vi "Frog generate Simu.vi"() -> ()   [LabVIEW 2024, in "File manipulate.lvclass"]
uses:
  File manipulate.lvclass
  File manipulate.lvclass/File manipulate.ctl
panel:
  in  "Transpose FROG Trace":bool
  out "temporal phase":cluster{"Y":dbl[], "Y":dbl[]}[](graph)
  in  "Save Fichier":bool
  in  "dispersive element":T1={"material"="BK7", "thickness"=0.0} {"thickness" format="%.2f"}
  out "Lambda":dbl[](array[numeric])=[479.83343142647254, 480.4599804843464, 481.0865295422202, 481.71307860009404, 482.33962765796787, 482.9661767158417, 483.59272577371553, 484.21927483158936, 484.8458238894632, 485.472372947337, 486.09892200521085, 486.7254710630847, 487.3520201209585, 487.97856917883234, 488.6051182367062, 489.23166729458, 489.85821635245384, 490.48476541032767, 491.1113144682015, 491.73786352607533, 492.36441258394916, 492.990961641823, 493.6175106996968, 494.24405975757065, 494.8706088154445, 495.4971578733183, 496.12370693119215, 496.750255989066, 497.3768050469398, 498.00335410481364, 498.62990316268747, 499.2564522205613, 499.88300127843513, 500.50955033630896, 501.1360993941828, 501.7626484520566, 502.38919750993045, 503.0157465678043, 503.6422956256781, 504.26884468355195, 504.8953937414258, 505.5219427992996, 506.14849185717344, 506.77504091504727, 507.4015899729211, 508.02813903079493, 508.65468808866876, 509.2812371465426, 509.9077862044164, 510.53433526229026, 511.1608843201641, 511.7874333780379, 512.4139824359117, 513.0405314937856, 513.6670805516594, 514.2936296095332, 514.9201786674071, 515.5467277252809, 516.1732767831547, 516.7998258410286, 517.4263748989024, 518.0529239567762, 518.6794730146501, 519.3060220725239, 519.9325711303977, 520.5591201882715, 521.1856692461454, 521.8122183040192, 522.438767361893, 523.0653164197669, 523.6918654776407, 524.3184145355145, 524.9449635933884, 525.5715126512622, 526.198061709136, 526.8246107670099, 527.4511598248837, 528.0777088827575, 528.7042579406314, 529.3308069985052, 529.957356056379, 530.5839051142528, 531.2104541721267, 531.8370032300005, 532.4635522878743, 533.0901013457482, 533.716650403622, 534.3431994614958, 534.9697485193697, 535.5962975772435, 536.2228466351173, 536.8493956929912, 537.475944750865, 538.1024938087388, 538.7290428666126, 539.3555919244865, 539.9821409823603, 540.6086900402341, 541.235239098108, 541.8617881559818, 542.4883372138556, 543.1148862717295, 543.7414353296033, 544.3679843874771, 544.994533445351, 545.6210825032248, 546.2476315610986, 546.8741806189724, 547.5007296768463, 548.1272787347201, 548.7538277925939, 549.3803768504678, 550.0069259083416, 550.6334749662154, 551.2600240240893, 551.8865730819631, 552.5131221398369, 553.1396711977108, 553.7662202555846, 554.3927693134584, 555.0193183713322, 555.6458674292061, 556.2724164870799, 556.8989655449537, 557.5255146028276, 558.1520636607014, 558.7786127185752, 559.4051617764491, 560.0317108343229, 560.6582598921967, 561.2848089500706, 561.9113580079444, 562.5379070658182, 563.164456123692, 563.7910051815659, 564.4175542394397, 565.0441032973135, 565.6706523551874, 566.2972014130612, 566.923750470935, 567.5502995288089, 568.1768485866827, 568.8033976445565, 569.4299467024304, 570.0564957603042, 570.683044818178, 571.3095938760518, 571.9361429339257, 572.5626919917995, 573.1892410496733, 573.8157901075472, 574.442339165421, 575.0688882232948, 575.6954372811687, 576.3219863390425, 576.9485353969163, 577.5750844547902, 578.201633512664, 578.8281825705378, 579.4547316284117, 580.0812806862855, 580.7078297441593, 581.3343788020331, 581.960927859907, 582.5874769177808, 583.2140259756546, 583.8405750335285, 584.4671240914023, 585.0936731492761, 585.72022220715, 586.3467712650238, 586.9733203228976, 587.5998693807715, 588.2264184386453, 588.8529674965191, 589.479516554393, 590.1060656122668, 590.7326146701406, 591.3591637280144, 591.9857127858883, 592.6122618437621, 593.2388109016359, 593.8653599595098, 594.4919090173836, 595.1184580752574, 595.7450071331313, 596.3715561910051, 596.9981052488789, 597.6246543067527, 598.2512033646266, 598.8777524225004, 599.5043014803742, 600.1308505382481, 600.7573995961219, 601.3839486539957, 602.0104977118696, 602.6370467697434, 603.2635958276172, 603.890144885491, 604.5166939433649, 605.1432430012387, 605.7697920591125, 606.3963411169864, 607.0228901748602, 607.649439232734, 608.2759882906079, 608.9025373484817, 609.5290864063555, 610.1556354642294, 610.7821845221032, 611.408733579977, 612.0352826378509, 612.6618316957247, 613.2883807535985, 613.9149298114723, 614.5414788693462, 615.16802792722, 615.7945769850938, 616.4211260429677, 617.0476751008415, 617.6742241587153, 618.3007732165892, 618.927322274463, 619.5538713323368, 620.1804203902107, 620.8069694480845, 621.4335185059583, 622.0600675638321, 622.686616621706, 623.3131656795798, 623.9397147374536, 624.5662637953275, 625.1928128532013, 625.8193619110751, 626.445910968949, 627.0724600268228, 627.6990090846966, 628.3255581425705, 628.9521072004443, 629.5786562583181, 630.205205316192, 630.8317543740658, 631.4583034319396, 632.0848524898134, 632.7114015476873, 633.3379506055611, 633.9644996634349, 634.5910487213088, 635.2175977791826, 635.8441468370564, 636.4706958949303, 637.0972449528041, 637.7237940106779, 638.3503430685518, 638.9768921264256, 639.6034411842994, 640.2299902421732, 640.8565393000471, 641.4830883579209, 642.1096374157947, 642.7361864736686, 643.3627355315424, 643.9892845894162, 644.6158336472901, 645.2423827051639, 645.8689317630377, 646.4954808209116, 647.1220298787854, 647.7485789366592, 648.375127994533, 649.0016770524069, 649.6282261102807, 650.2547751681545, 650.8813242260284, 651.5078732839022, 652.134422341776, 652.7609713996499, 653.3875204575237, 654.0140695153975, 654.6406185732714, 655.2671676311452, 655.893716689019, 656.5202657468928, 657.1468148047667, 657.7733638626405, 658.3999129205143, 659.0264619783882, 659.653011036262, 660.2795600941358, 660.9061091520097, 661.5326582098835, 662.1592072677573, 662.7857563256312, 663.412305383505, 664.0388544413788, 664.6654034992526, 665.2919525571265, 665.9185016150003, 666.5450506728741, 667.171599730748, 667.7981487886218, 668.4246978464956, 669.0512469043695, 669.6777959622433, 670.3043450201171, 670.930894077991, 671.5574431358648, 672.1839921937386, 672.8105412516124, 673.4370903094863, 674.0636393673601, 674.6901884252339, 675.3167374831078, 675.9432865409816, 676.5698355988554, 677.1963846567293, 677.8229337146031, 678.4494827724769, 679.0760318303508, 679.7025808882246, 680.3291299460984, 680.9556790039723, 681.5822280618461, 682.2087771197199, 682.8353261775937, 683.4618752354676, 684.0884242933414, 684.7149733512152, 685.3415224090891, 685.9680714669629, 686.5946205248367, 687.2211695827106, 687.8477186405844, 688.4742676984582, 689.100816756332, 689.7273658142059, 690.3539148720797, 690.9804639299535, 691.6070129878274, 692.2335620457012, 692.860111103575, 693.4866601614489, 694.1132092193227, 694.7397582771965, 695.3663073350704, 695.9928563929442, 696.619405450818, 697.2459545086919, 697.8725035665657, 698.4990526244395, 699.1256016823133, 699.7521507401872, 700.378699798061, 701.0052488559348, 701.6317979138087, 702.2583469716825, 702.8848960295563, 703.5114450874302, 704.137994145304, 704.7645432031778, 705.3910922610517, 706.0176413189255, 706.6441903767993, 707.2707394346731, 707.897288492547, 708.5238375504208, 709.1503866082946, 709.7769356661685, 710.4034847240423, 711.0300337819161, 711.65658283979, 712.2831318976638, 712.9096809555376, 713.5362300134115, 714.1627790712853, 714.7893281291591, 715.415877187033, 716.0424262449068, 716.6689753027806, 717.2955243606544, 717.9220734185283, 718.5486224764021, 719.1751715342759, 719.8017205921498, 720.4282696500236, 721.0548187078974, 721.6813677657713, 722.3079168236451, 722.9344658815189, 723.5610149393927, 724.1875639972666, 724.8141130551404, 725.4406621130142, 726.0672111708881, 726.6937602287619, 727.3203092866357, 727.9468583445096, 728.5734074023834, 729.1999564602572, 729.8265055181311, 730.4530545760049, 731.0796036338787, 731.7061526917525, 732.3327017496264, 732.9592508075002, 733.585799865374, 734.2123489232479, 734.8388979811217, 735.4654470389955, 736.0919960968694, 736.7185451547432, 737.345094212617, 737.9716432704909, 738.5981923283647, 739.2247413862385, 739.8512904441124, 740.4778395019862, 741.10438855986, 741.7309376177338, 742.3574866756077, 742.9840357334815, 743.6105847913553, 744.2371338492292, 744.863682907103, 745.4902319649768, 746.1167810228507, 746.7433300807245, 747.3698791385983, 747.9964281964722, 748.622977254346, 749.2495263122198, 749.8760753700936, 750.5026244279675, 751.1291734858413, 751.7557225437151, 752.382271601589, 753.0088206594628, 753.6353697173366, 754.2619187752105, 754.8884678330843, 755.5150168909581, 756.141565948832, 756.7681150067058, 757.3946640645796, 758.0212131224534, 758.6477621803273, 759.2743112382011, 759.9008602960749, 760.5274093539488, 761.1539584118226, 761.7805074696964, 762.4070565275703, 763.0336055854441, 763.6601546433179, 764.2867037011918, 764.9132527590656, 765.5398018169394, 766.1663508748132, 766.7928999326871, 767.4194489905609, 768.0459980484347, 768.6725471063086, 769.2990961641824, 769.9256452220562, 770.5521942799301, 771.1787433378039, 771.8052923956777, 772.4318414535516, 773.0583905114254, 773.6849395692992, 774.311488627173, 774.9380376850469, 775.5645867429207, 776.1911358007945, 776.8176848586684, 777.4442339165422, 778.070782974416, 778.6973320322899, 779.3238810901637, 779.9504301480375, 780.5769792059114, 781.2035282637852, 781.830077321659, 782.4566263795328, 783.0831754374067, 783.7097244952805, 784.3362735531543, 784.9628226110282, 785.589371668902, 786.2159207267758, 786.8424697846497, 787.4690188425235, 788.0955679003973, 788.7221169582712, 789.348666016145, 789.9752150740188, 790.6017641318927, 791.2283131897665, 791.8548622476403, 792.4814113055141, 793.107960363388, 793.7345094212618, 794.3610584791356, 794.9876075370095, 795.6141565948833, 796.2407056527571, 796.867254710631, 797.4938037685048, 798.1203528263786, 798.7469018842525, 799.3734509421263, 800.0000000000001, 800.626549057874, 801.2530981157478, 801.8796471736216, 802.5061962314954, 803.1327452893693, 803.7592943472431, 804.3858434051169, 805.0123924629908, 805.6389415208646, 806.2654905787384, 806.8920396366123, 807.5185886944861, 808.1451377523599, 808.7716868102337, 809.3982358681076, 810.0247849259814, 810.6513339838552, 811.2778830417291, 811.9044320996029, 812.5309811574767, 813.1575302153506, 813.7840792732244, 814.4106283310982, 815.037177388972, 815.6637264468459, 816.2902755047197, 816.9168245625935, 817.5433736204674, 818.1699226783412, 818.796471736215, 819.4230207940889, 820.0495698519627, 820.6761189098365, 821.3026679677104, 821.9292170255842, 822.555766083458, 823.1823151413319, 823.8088641992057, 824.4354132570795, 825.0619623149533, 825.6885113728272, 826.315060430701, 826.9416094885748, 827.5681585464487, 828.1947076043225, 828.8212566621963, 829.4478057200702, 830.074354777944, 830.7009038358178, 831.3274528936917, 831.9540019515655, 832.5805510094393, 833.2071000673131, 833.833649125187, 834.4601981830608, 835.0867472409346, 835.7132962988085, 836.3398453566823, 836.9663944145561, 837.59294347243, 838.2194925303038, 838.8460415881776, 839.4725906460515, 840.0991397039253, 840.7256887617991, 841.352237819673, 841.9787868775468, 842.6053359354206, 843.2318849932944, 843.8584340511683, 844.4849831090421, 845.1115321669159, 845.7380812247898, 846.3646302826636, 846.9911793405374, 847.6177283984113, 848.2442774562851, 848.8708265141589, 849.4973755720328, 850.1239246299066, 850.7504736877804, 851.3770227456542, 852.0035718035281, 852.6301208614019, 853.2566699192757, 853.8832189771496, 854.5097680350234, 855.1363170928972, 855.7628661507711, 856.3894152086449, 857.0159642665187, 857.6425133243926, 858.2690623822664, 858.8956114401402, 859.522160498014, 860.1487095558879, 860.7752586137617, 861.4018076716355, 862.0283567295094, 862.6549057873832, 863.281454845257, 863.9080039031309, 864.5345529610047, 865.1611020188785, 865.7876510767524, 866.4142001346262, 867.0407491925, 867.6672982503738, 868.2938473082477, 868.9203963661215, 869.5469454239953, 870.1734944818692, 870.800043539743, 871.4265925976168, 872.0531416554907, 872.6796907133645, 873.3062397712383, 873.9327888291122, 874.559337886986, 875.1858869448598, 875.8124360027336, 876.4389850606075, 877.0655341184813, 877.6920831763551, 878.318632234229, 878.9451812921028, 879.5717303499766, 880.1982794078505, 880.8248284657243, 881.4513775235981, 882.077926581472, 882.7044756393458, 883.3310246972196, 883.9575737550934, 884.5841228129673, 885.2106718708411, 885.8372209287149, 886.4637699865888, 887.0903190444626, 887.7168681023364, 888.3434171602103, 888.9699662180841, 889.5965152759579, 890.2230643338318, 890.8496133917056, 891.4761624495794, 892.1027115074533, 892.7292605653271, 893.3558096232009, 893.9823586810747, 894.6089077389486, 895.2354567968224, 895.8620058546962, 896.4885549125701, 897.1151039704439, 897.7416530283177, 898.3682020861916, 898.9947511440654, 899.6213002019392, 900.247849259813, 900.8743983176869, 901.5009473755607, 902.1274964334345, 902.7540454913084, 903.3805945491822, 904.007143607056, 904.6336926649299, 905.2602417228037, 905.8867907806775, 906.5133398385514, 907.1398888964252, 907.766437954299, 908.3929870121729, 909.0195360700467, 909.6460851279205, 910.2726341857943, 910.8991832436682, 911.525732301542, 912.1522813594158, 912.7788304172897, 913.4053794751635, 914.0319285330373, 914.6584775909112, 915.285026648785, 915.9115757066588, 916.5381247645327, 917.1646738224065, 917.7912228802803, 918.4177719381541, 919.044320996028, 919.6708700539018, 920.2974191117756, 920.9239681696495, 921.5505172275233, 922.1770662853971, 922.803615343271, 923.4301644011448, 924.0567134590186, 924.6832625168925, 925.3098115747663, 925.9363606326401, 926.562909690514, 927.1894587483878, 927.8160078062616, 928.4425568641354, 929.0691059220093, 929.6956549798831, 930.3222040377569, 930.9487530956308, 931.5753021535046, 932.2018512113784, 932.8284002692523, 933.4549493271261, 934.0814983849999, 934.7080474428737, 935.3345965007476, 935.9611455586214, 936.5876946164952, 937.2142436743691, 937.8407927322429, 938.4673417901167, 939.0938908479906, 939.7204399058644, 940.3469889637382, 940.9735380216121, 941.6000870794859, 942.2266361373597, 942.8531851952336, 943.4797342531074, 944.1062833109812, 944.732832368855, 945.3593814267289, 945.9859304846027, 946.6124795424765, 947.2390286003504, 947.8655776582242, 948.492126716098, 949.1186757739719, 949.7452248318457, 950.3717738897195, 950.9983229475934, 951.6248720054672, 952.251421063341, 952.8779701212148, 953.5045191790887, 954.1310682369625, 954.7576172948363, 955.3841663527102, 956.010715410584, 956.6372644684578, 957.2638135263317, 957.8903625842055, 958.5169116420793, 959.1434606999532, 959.770009757827, 960.3965588157008, 961.0231078735746, 961.6496569314485, 962.2762059893223, 962.9027550471961, 963.52930410507, 964.1558531629438, 964.7824022208176, 965.4089512786915, 966.0355003365653, 966.6620493944391, 967.288598452313, 967.9151475101868, 968.5416965680606, 969.1682456259344, 969.7947946838083, 970.4213437416821, 971.0478927995559, 971.6744418574298, 972.3009909153036, 972.9275399731774, 973.5540890310513, 974.1806380889251, 974.8071871467989, 975.4337362046728, 976.0602852625466, 976.6868343204204, 977.3133833782942, 977.9399324361681, 978.5664814940419, 979.1930305519157, 979.8195796097896, 980.4461286676634, 981.0726777255372, 981.6992267834111, 982.3257758412849, 982.9523248991587, 983.5788739570326, 984.2054230149064, 984.8319720727802, 985.458521130654, 986.0850701885279, 986.7116192464017, 987.3381683042755, 987.9647173621494, 988.5912664200232, 989.217815477897, 989.8443645357709, 990.4709135936447, 991.0974626515185, 991.7240117093924, 992.3505607672662, 992.97710982514, 993.6036588830138, 994.2302079408877, 994.8567569987615, 995.4833060566353, 996.1098551145092, 996.736404172383, 997.3629532302568, 997.9895022881307, 998.6160513460045, 999.2426004038783, 999.8691494617522, 1000.495698519626, 1001.1222475774998, 1001.7487966353737, 1002.3753456932475, 1003.0018947511213, 1003.6284438089951, 1004.254992866869, 1004.8815419247428, 1005.5080909826166, 1006.1346400404905, 1006.7611890983643, 1007.3877381562381, 1008.014287214112, 1008.6408362719858, 1009.2673853298596, 1009.8939343877335, 1010.5204834456073, 1011.1470325034811, 1011.773581561355, 1012.4001306192288, 1013.0266796771026, 1013.6532287349764, 1014.2797777928503, 1014.9063268507241, 1015.5328759085979, 1016.1594249664718, 1016.7859740243456, 1017.4125230822194, 1018.0390721400933, 1018.6656211979671, 1019.2921702558409, 1019.9187193137147, 1020.5452683715886, 1021.1718174294624, 1021.7983664873362, 1022.4249155452101, 1023.0514646030839, 1023.6780136609577, 1024.3045627188317, 1024.9311117767054, 1025.557660834579, 1026.184209892453, 1026.810758950327, 1027.4373080082007, 1028.0638570660744, 1028.6904061239484, 1029.3169551818223, 1029.943504239696, 1030.5700532975698, 1031.1966023554437, 1031.8231514133176, 1032.4497004711914, 1033.076249529065, 1033.702798586939, 1034.329347644813, 1034.9558967026867, 1035.5824457605604, 1036.2089948184343, 1036.8355438763083, 1037.462092934182, 1038.0886419920557, 1038.7151910499297, 1039.3417401078036, 1039.9682891656773, 1040.594838223551, 1041.221387281425, 1041.847936339299, 1042.4744853971727, 1043.1010344550464, 1043.7275835129203, 1044.3541325707943, 1044.980681628668, 1045.6072306865417, 1046.2337797444156, 1046.8603288022896, 1047.4868778601633, 1048.113426918037, 1048.739975975911, 1049.366525033785, 1049.9930740916586, 1050.6196231495323, 1051.2461722074063, 1051.8727212652802, 1052.499270323154, 1053.1258193810277, 1053.7523684389016, 1054.3789174967756, 1055.0054665546493, 1055.632015612523, 1056.258564670397, 1056.8851137282709, 1057.5116627861446, 1058.1382118440183, 1058.7647609018923, 1059.3913099597662, 1060.01785901764, 1060.6444080755136, 1061.2709571333876, 1061.8975061912615, 1062.5240552491352, 1063.150604307009, 1063.777153364883, 1064.4037024227569, 1065.0302514806306, 1065.6568005385043, 1066.2833495963782, 1066.9098986542522, 1067.536447712126, 1068.1629967699996, 1068.7895458278736, 1069.4160948857475, 1070.0426439436212, 1070.669193001495, 1071.2957420593689, 1071.9222911172428, 1072.5488401751165, 1073.1753892329903, 1073.8019382908642, 1074.4284873487381, 1075.0550364066119, 1075.6815854644856, 1076.3081345223595, 1076.9346835802335, 1077.5612326381072, 1078.187781695981, 1078.8143307538548, 1079.4408798117288, 1080.0674288696025, 1080.6939779274762, 1081.3205269853502, 1081.9470760432241, 1082.5736251010978, 1083.2001741589715, 1083.8267232168455, 1084.4532722747194, 1085.0798213325932, 1085.7063703904669, 1086.3329194483408, 1086.9594685062148, 1087.5860175640885, 1088.2125666219622, 1088.8391156798361, 1089.46566473771, 1090.0922137955838, 1090.7187628534575, 1091.3453119113315, 1091.9718609692054, 1092.5984100270791, 1093.2249590849528, 1093.8515081428268, 1094.4780572007007, 1095.1046062585744, 1095.7311553164482, 1096.357704374322, 1096.984253432196, 1097.6108024900698, 1098.2373515479435, 1098.8639006058174, 1099.4904496636914, 1100.116998721565, 1100.7435477794388, 1101.3700968373128, 1101.9966458951867, 1102.6231949530604, 1103.2497440109341, 1103.876293068808, 1104.502842126682, 1105.1293911845557, 1105.7559402424295, 1106.3824893003034, 1107.0090383581773, 1107.635587416051, 1108.2621364739248, 1108.8886855317987, 1109.5152345896727, 1110.1417836475464, 1110.76833270542, 1111.394881763294, 1112.021430821168, 1112.6479798790417, 1113.2745289369154, 1113.9010779947894, 1114.5276270526633, 1115.154176110537, 1115.7807251684108, 1116.4072742262847, 1117.0338232841586, 1117.6603723420324, 1118.286921399906, 1118.91347045778, 1119.540019515654, 1120.1665685735277, 1120.7931176314014]
  out "dt":dbl=6.669999999999959
  out "dl":dbl=0.6265490578738309
  out "l0":dbl=479.83343142647254
  in  "Gauss (temporal)":T2={"energy"=0.001, "beam diameter"=0.001, "l0"=8.000000000000001e-07, "Dt"=3.0000000000000005e-14} {"beam diameter" format="%.2f"; "Dt" format="%.2f"; "l0" format="%.2f"; "energy" format="%.2f"}
  in  "sampling":T3={"resolution"=enum."high spectral", "2^n"=0, "tmax"=1e-12} {"tmax" format="%#_6f"}
  out "spectral phase":cluster{"Y":dbl[], "Y":dbl[]}[](graph)=[{"Y"=[-0.17112071020073646, -0.16895462526148664, -0.1667885403222368, -0.16462245538298698, -0.16245637044373715, -0.16029028550448732, -0.1581242005652375, -0.15595811562598766, -0.15379203068673786, -0.151625945747488, -0.1494598608082382, -0.14729377586898834, -0.14512769092973854, -0.14296160599048868, -0.14079552105123888, -0.13862943611198902, -0.1364633511727392, -0.13429726623348937, -0.13213118129423954, -0.1299650963549897, -0.12779901141573988, -0.12563292647649008, -0.12346684153724023, -0.1213007565979904, -0.11913467165874057, -0.11696858671949074, -0.11480250178024093, -0.1126364168409911, -0.11047033190174127, -0.10830424696249144, -0.10613816202324161, -0.10397207708399178, -0.10180599214474194, -0.09963990720549211, -0.09747382226624228, -0.09530773732699245, -0.09314165238774262, -0.09097556744849279, -0.08880948250924296, -0.08664339756999315, -0.08447731263074332, -0.08231122769149349, -0.08014514275224366, -0.07797905781299383, -0.075812972873744, -0.07364688793449417, -0.07148080299524434, -0.06931471805599451, -0.06714863311674468, -0.06498254817749485, -0.06281646323824504, -0.0606503782989952, -0.05848429335974537, -0.05631820842049555, -0.05415212348124572, -0.05198603854199589, -0.049819953602746055, -0.047653868663496225, -0.045487783724246396, -0.04332169878499657, -0.041155613845746744, -0.038989528906496915, -0.036823443967247085, -0.034657359027997256, -0.03249127408874743, -0.0303251891494976, -0.028159104210247775, -0.025993019270997945, -0.023826934331748113, -0.021660849392498287, -0.019494764453248457, -0.017328679513998628, -0.0151625945747488, -0.012996509635498973, -0.010830424696249143, -0.008664339756999314, -0.006498254817749486, -0.004332169878499657, -0.0021660849392498285, 0.0, 0.0021660849392498285, 0.004332169878499657, 0.006498254817749486, 0.008664339756999314, 0.010830424696249143, 0.012996509635498973, 0.0151625945747488, 0.017328679513998628, 0.019494764453248457, 0.021660849392498287, 0.023826934331748113, 0.025993019270997945, 0.028159104210247775, 0.0303251891494976, 0.03249127408874743, 0.034657359027997256, 0.036823443967247085, 0.038989528906496915, 0.041155613845746744, 0.04332169878499657, 0.045487783724246396, 0.047653868663496225, 0.049819953602746055, 0.05198603854199589, 0.05415212348124572, 0.05631820842049555, 0.05848429335974537, 0.0606503782989952, 0.06281646323824504, 0.06498254817749485, 0.06714863311674468, 0.06931471805599451, 0.07148080299524434, 0.07364688793449417, 0.075812972873744, 0.07797905781299383, 0.08014514275224366, 0.08231122769149349, 0.08447731263074332, 0.08664339756999315, 0.08880948250924296, 0.09097556744849279, 0.09314165238774262, 0.09530773732699245, 0.09747382226624228, 0.09963990720549211, 0.10180599214474194, 0.10397207708399178, 0.10613816202324161, 0.10830424696249144, 0.11047033190174127, 0.1126364168409911, 0.11480250178024093, 0.11696858671949074, 0.11913467165874057, 0.1213007565979904, 0.12346684153724023, 0.12563292647649008, 0.12779901141573988, 0.1299650963549897, 0.13213118129423954, 0.13429726623348937, 0.1364633511727392, 0.13862943611198902, 0.14079552105123888, 0.14296160599048868, 0.14512769092973854, 0.14729377586898834, 0.1494598608082382, 0.151625945747488, 0.15379203068673786, 0.15595811562598766, 0.1581242005652375, 0.16029028550448732, 0.16245637044373715, 0.16462245538298698, 0.1667885403222368, 0.16895462526148664], "Y"=[-31.17319838706582, -28.41009212549852, -25.72156616547755, -23.106604196419145, -20.564189907739806, -18.093306988855804, -15.692939129184245, -13.362070018141393, -11.099683345143523, -8.904762799607694, -6.7762920709501895, -4.713254848587267, -2.714634821936001, -0.7794156804126388, 1.0934188865662493, 2.9048851895843355, 4.655999539224675, 6.347778246070939, 7.98123762070677, 9.55739397371526, 11.077263615680074, 12.54186285718482, 13.952208008812615, 15.309315381147115, 16.614201284771923, 17.867882030270206, 19.07137392822556, 20.2256932892216, 21.331856423841504, 22.390879642668896, 23.403779256287322, 24.37157157528002, 25.295272910230583, 26.17589957172256, 27.01446787033912, 27.811994116664117, 28.56949462128081, 29.287985694772498, 29.96848364772298, 30.612004790715552, 31.219565434333525, 31.792181889160656, 32.33087046578026, 32.83664747477569, 33.31052922673063, 33.75353203222843, 34.16667220185246, 34.550966046186375, 34.907429875813534, 35.23708000131733, 35.54093273328137, 35.820004382289056, 36.075311258923776, 36.30786967376912, 36.51869593740848, 36.70880636042529, 36.87921725340309, 37.030944926925294, 37.165005691575345, 37.28241585793676, 37.384191736592975, 37.47134963812743, 37.544905873123625, 37.605876752164995, 37.65527858583502, 37.69412768471716, 37.723440359394864, 37.74423292045161, 37.757521678470845, 37.764322944036046, 37.765653027730664, 37.762528240138174, 37.75596489184203, 37.74697929342568, 37.73658775547261, 37.72580658856628, 37.71565210329014, 37.707140610227654, 37.701288419962296, 37.69911184307752, 37.701627190156785, 37.70985077178356, 37.7247988985413, 37.74748788101348, 37.77893402978354, 37.82015365543497, 37.87216306855122, 37.93597857971574, 38.012616499512006, 38.10309313852349, 38.20842480733362, 38.3296278165259, 38.46771847668378, 38.623713098390674, 38.798627992230124, 38.99347946878556, 39.20928383864039, 39.44705741237817, 39.70781650058226, 39.99257741383624, 40.302356462723516, 40.638169957827465, 41.001034209731706, 41.391965529019636, 41.81198022627461, 42.26209461208028, 42.743324997020025, 43.25668769167718, 43.803199006635445, 44.38387525247816, 44.99973273978866, 45.65178777915067, 46.34105668114753, 47.06855575636253, 47.83530131537945, 48.64230966878161, 49.49059712715226, 50.381180001075265, 51.31507460113388, 52.293297237911354, 53.316864221991594, 54.38679186395783, 55.50409647439328, 56.66979436388192, 57.88490184300694, 59.15043522235153, 60.467410812499715, 61.83684492403469, 63.25975386753958, 64.7371539535985, 66.27006149279457, 67.8594927957109, 69.5064641729317, 71.21199193504005, 72.97709239261901, 74.80278185625285, 76.69007663652418, 78.63999304401736, 80.6535473893154, 82.7317559830013, 84.87563513565945, 87.08620115787285, 89.36447036022444, 91.71145905329873, 94.12818354767866, 96.61566015394712, 99.17490518268875, 101.80693494448637, 104.51276574992285, 107.29341390958291, 110.14989573404938, 113.08322753390505, 109.81124031255516, 112.90132099494164, 109.78811527728809, 113.03901008453856, 110.08865111291661, 107.22123998018455]}, {"Y"=[-0.17112071020073646, -0.16895462526148664, -0.1667885403222368, -0.16462245538298698, -0.16245637044373715, -0.16029028550448732, -0.1581242005652375, -0.15595811562598766, -0.15379203068673786, -0.151625945747488, -0.1494598608082382, -0.14729377586898834, -0.14512769092973854, -0.14296160599048868, -0.14079552105123888, -0.13862943611198902, -0.1364633511727392, -0.13429726623348937, -0.13213118129423954, -0.1299650963549897, -0.12779901141573988, -0.12563292647649008, -0.12346684153724023, -0.1213007565979904, -0.11913467165874057, -0.11696858671949074, -0.11480250178024093, -0.1126364168409911, -0.11047033190174127, -0.10830424696249144, -0.10613816202324161, -0.10397207708399178, -0.10180599214474194, -0.09963990720549211, -0.09747382226624228, -0.09530773732699245, -0.09314165238774262, -0.09097556744849279, -0.08880948250924296, -0.08664339756999315, -0.08447731263074332, -0.08231122769149349, -0.08014514275224366, -0.07797905781299383, -0.075812972873744, -0.07364688793449417, -0.07148080299524434, -0.06931471805599451, -0.06714863311674468, -0.06498254817749485, -0.06281646323824504, -0.0606503782989952, -0.05848429335974537, -0.05631820842049555, -0.05415212348124572, -0.05198603854199589, -0.049819953602746055, -0.047653868663496225, -0.045487783724246396, -0.04332169878499657, -0.041155613845746744, -0.038989528906496915, -0.036823443967247085, -0.034657359027997256, -0.03249127408874743, -0.0303251891494976, -0.028159104210247775, -0.025993019270997945, -0.023826934331748113, -0.021660849392498287, -0.019494764453248457, -0.017328679513998628, -0.0151625945747488, -0.012996509635498973, -0.010830424696249143, -0.008664339756999314, -0.006498254817749486, -0.004332169878499657, -0.0021660849392498285, 0.0, 0.0021660849392498285, 0.004332169878499657, 0.006498254817749486, 0.008664339756999314, 0.010830424696249143, 0.012996509635498973, 0.0151625945747488, 0.017328679513998628, 0.019494764453248457, 0.021660849392498287, 0.023826934331748113, 0.025993019270997945, 0.028159104210247775, 0.0303251891494976, 0.03249127408874743, 0.034657359027997256, 0.036823443967247085, 0.038989528906496915, 0.041155613845746744, 0.04332169878499657, 0.045487783724246396, 0.047653868663496225, 0.049819953602746055, 0.05198603854199589, 0.05415212348124572, 0.05631820842049555, 0.05848429335974537, 0.0606503782989952, 0.06281646323824504, 0.06498254817749485, 0.06714863311674468, 0.06931471805599451, 0.07148080299524434, 0.07364688793449417, 0.075812972873744, 0.07797905781299383, 0.08014514275224366, 0.08231122769149349, 0.08447731263074332, 0.08664339756999315, 0.08880948250924296, 0.09097556744849279, 0.09314165238774262, 0.09530773732699245, 0.09747382226624228, 0.09963990720549211, 0.10180599214474194, 0.10397207708399178, 0.10613816202324161, 0.10830424696249144, 0.11047033190174127, 0.1126364168409911, 0.11480250178024093, 0.11696858671949074, 0.11913467165874057, 0.1213007565979904, 0.12346684153724023, 0.12563292647649008, 0.12779901141573988, 0.1299650963549897, 0.13213118129423954, 0.13429726623348937, 0.1364633511727392, 0.13862943611198902, 0.14079552105123888, 0.14296160599048868, 0.14512769092973854, 0.14729377586898834, 0.1494598608082382, 0.151625945747488, 0.15379203068673786, 0.15595811562598766, 0.1581242005652375, 0.16029028550448732, 0.16245637044373715, 0.16462245538298698, 0.1667885403222368, 0.16895462526148664], "Y"=[-32.85653058116809, -29.831240282503238, -26.898514859158446, -24.056707184503587, -21.304179529324443, -18.63930356182282, -16.060460347616477, -13.566040349739156, -11.154443428640567, -8.824078842186296, -6.573365245658064, -4.400730691753406, -2.3046126305859636, -0.28345790968515683, 1.6642772260033905, 3.5401271341182845, 5.345616774882063, 7.082261711101298, 8.751568108166628, 10.35503273405273, 11.894142959318273, 13.37037675710597, 14.78520270314261, 16.140079975738953, 17.436458355789807, 18.675778226774046, 19.85947057475452, 20.98895698837818, 22.065649658875962, 23.09095138006282, 24.06625554833779, 24.992946162683893, 25.87239782466822, 26.705975738441875, 27.495035710739984, 28.240924150881728, 28.9449780707703, 29.60852508489295, 30.232883410320927, 30.81936186670954, 31.36925987629812, 31.88386746391002, 32.36446525695264, 32.81232448541741, 33.22870698187979, 33.61486518149926, 33.97204212201937, 34.30147144376763, 34.60437738965567, 34.88197480517908, 35.13546913841753, 35.36605644003468, 35.57492336327828, 35.76324716398005, 35.93219570055578, 36.082927434005285, 36.2165914279124, 36.334327348444994, 36.437265464355, 36.52652664697834, 36.60322237023498, 36.66845471062893, 36.72331634724824, 36.76889056176496, 36.8062512384352, 36.83646286409909, 36.86058052818078, 36.8796499226885, 36.894707342214446, 36.906779683934886, 36.91688444761012, 36.92602973558448, 36.935214252786295, 36.945427306727986, 36.957648807505954, 36.97284926780065, 36.991989802876574, 37.016022130582236, 37.045888571350176, 37.082522048196985, 37.126846086723276, 37.179774815113696, 37.24221296413691, 37.31505586714564, 37.39918946007662, 37.495490281450635, 37.60482547237248, 37.728052776531, 37.86602054019905, 38.01956771223355, 38.189523844075424, 38.37670908974965, 38.5819342058652, 38.80600055161513, 39.04970008877648, 39.31381538171037, 39.59911959736192, 39.90637650526026, 40.23634047751862, 40.5897564888342, 40.96736011648826, 41.369877540346074, 41.79802554285698, 42.25251150905433, 42.734033426555484, 43.24327988556188, 43.780930078858965, 44.34765380181619, 44.9441114523871, 45.57095403110922, 46.228823141104115, 46.918350988077414, 47.640160380318754, 48.3948647287018, 49.18306804668425, 50.00536495030786, 50.86234065819838, 51.75457099156559, 52.682622374203376, 53.647051832489566, 54.64840699538604, 55.68722609443877, 56.76403796377768, 57.87936204011678, 59.0337083627541, 60.22757757357167, 61.4614609170356, 62.73584024019601, 64.05118799268706, 65.40796722672691, 66.80663159711777, 68.24762536124592, 69.73138337908163, 71.25833111317921, 72.828884628677, 74.44345059329738, 76.10242627734678, 77.80619955371563, 79.55514889787835, 81.34964338789352, 83.19004270440367, 85.07669713063531, 87.0099475523991, 88.99012545808965, 91.01755293868565, 93.09254268774973, 95.21539800142872, 97.38641277845328, 99.6058715201383, 101.87404933038249, 104.19121191566884, 106.55761558506413, 108.97350725021934, 111.43912442536941, 113.95469522733335, 116.52043837551412, 119.13656319189884, 121.80326960105853]}]
  in  "save option":T4(ring)
  in  "path to file":path=path "C:/Users/flepetit/Desktop/Labview Lab2"
  out "FWHM":dbl[unit]=6.492451086910603e-14 format="%.1f"
  out "temporal intensity":T5(graph)
  out "spectral phase\ntaylor coefficients [fs^n]":dbl[](array[numeric])=[37.082522048196985, 18.616822978824477, 1639.2731119297016, 90408.0807167296, -426880.6999661568] format="%.2e"
  in  "what":T6(ring)=enum."quadratic phase"
  out "SHG Frog":dbl[][](graph)
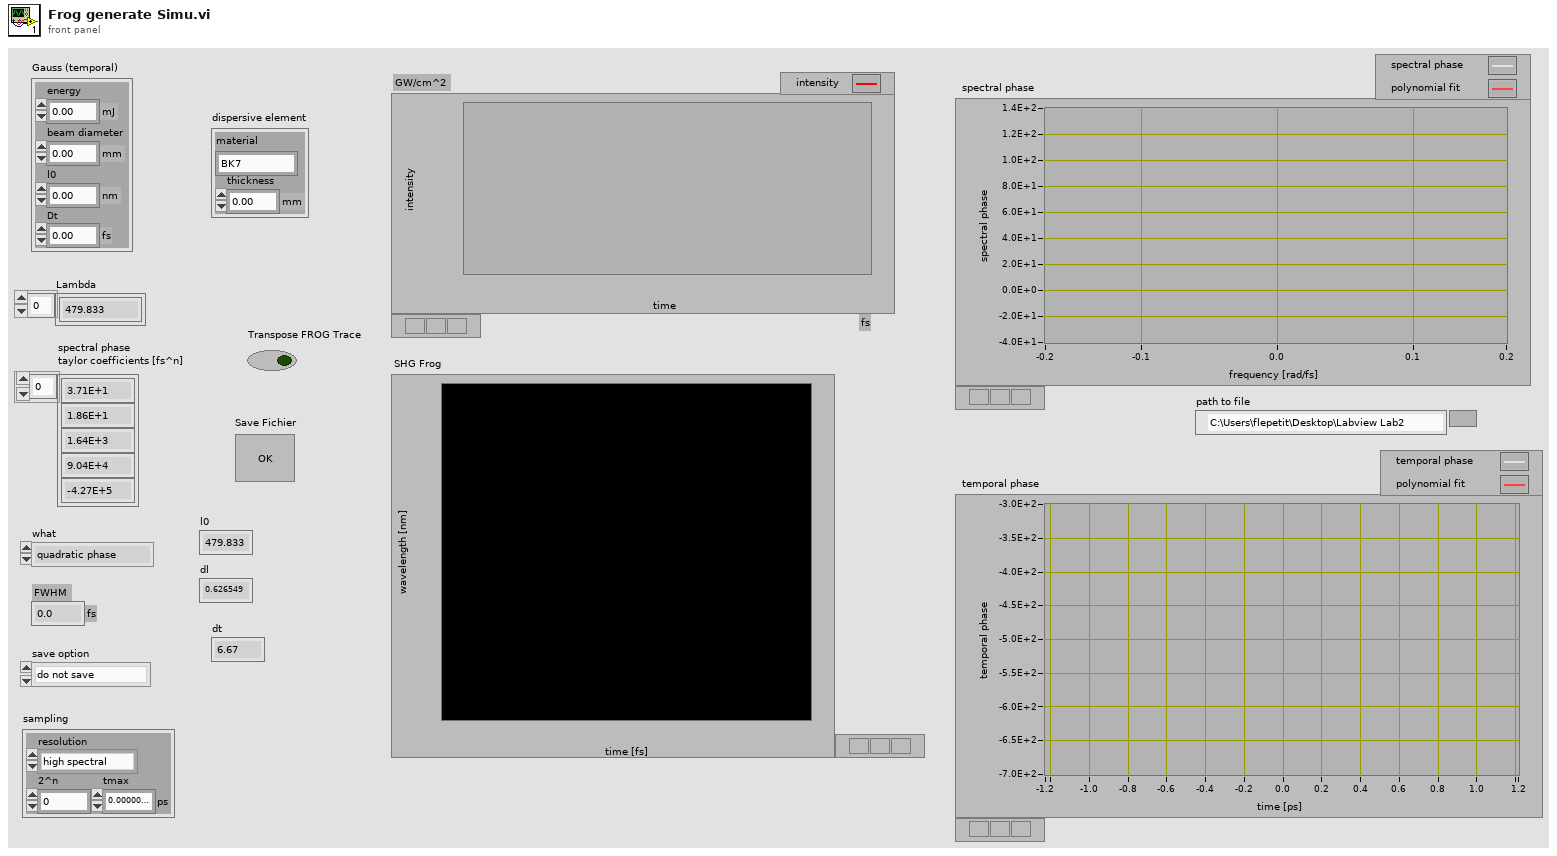
[diagram p1: front panel]
types:
  T1 = cluster{"material":string, "thickness":dbl[unit]}
  T2 = cluster{"energy":dbl[unit], "beam diameter":dbl[unit], "l0":dbl[unit], "Dt":dbl[unit]}
  T3 = cluster{"resolution":enum16{"high spectral", "balanced", "high temporal", "time window"}, "2^n":i32, "tmax":dbl[unit]}
  T4 = enum16{"do not save", "save jpeg", "save retrieval format"}
  T5 = cluster{"time":dbl[unit][], "intensity with units":dbl[unit][]}
  T6 = enum16{"no phase", "quadratic phase", "cubic phase", "quartic phase", "SPM", "double pulse", "double pulse pi"}
  T7 = cluster{"type":enum16{"SHG", "THG", "PG", "TG", "SD"}, "field size":enum16{"32x32", "64x64", "128x128", "256x256", "512x512", "1024x1024"}, "time step":dbl[unit], "save option":enum16{"do not save", "save jpeg", "save retrieval format"}, "path to file":path}
  T8 = typedef "pulse cluster.ctl" = cluster{"nop":i32, "auto":bool, "fluence":dbl[unit], "diameter":dbl[unit], "w0":dbl[unit], "t0":dbl[unit], "w":dbl[unit][], "|E(w)|":dbl[], "phi(w)":dbl[]}
  T9 = cluster{"type":enum16{"none", "interpolate", "arbitrary", "Taylor", "sinusoidal", "square", "sawtooth"}, "Taylor [fs^n]":dbl[], "periodic functions":cluster{"amplitude":dbl, "offset":dbl, "dt":dbl[unit], "phase":dbl}}
  T10 = cluster{"type":enum16{"none", "interpolate", "arbitrary", "Taylor", "sinusoidal", "square", "sawtooth"}, "Taylor [fs^n]":dbl[], "periodic functions 2":cluster{"amplitude":dbl, "offset":dbl, "dt":dbl[unit], "phase":dbl}}
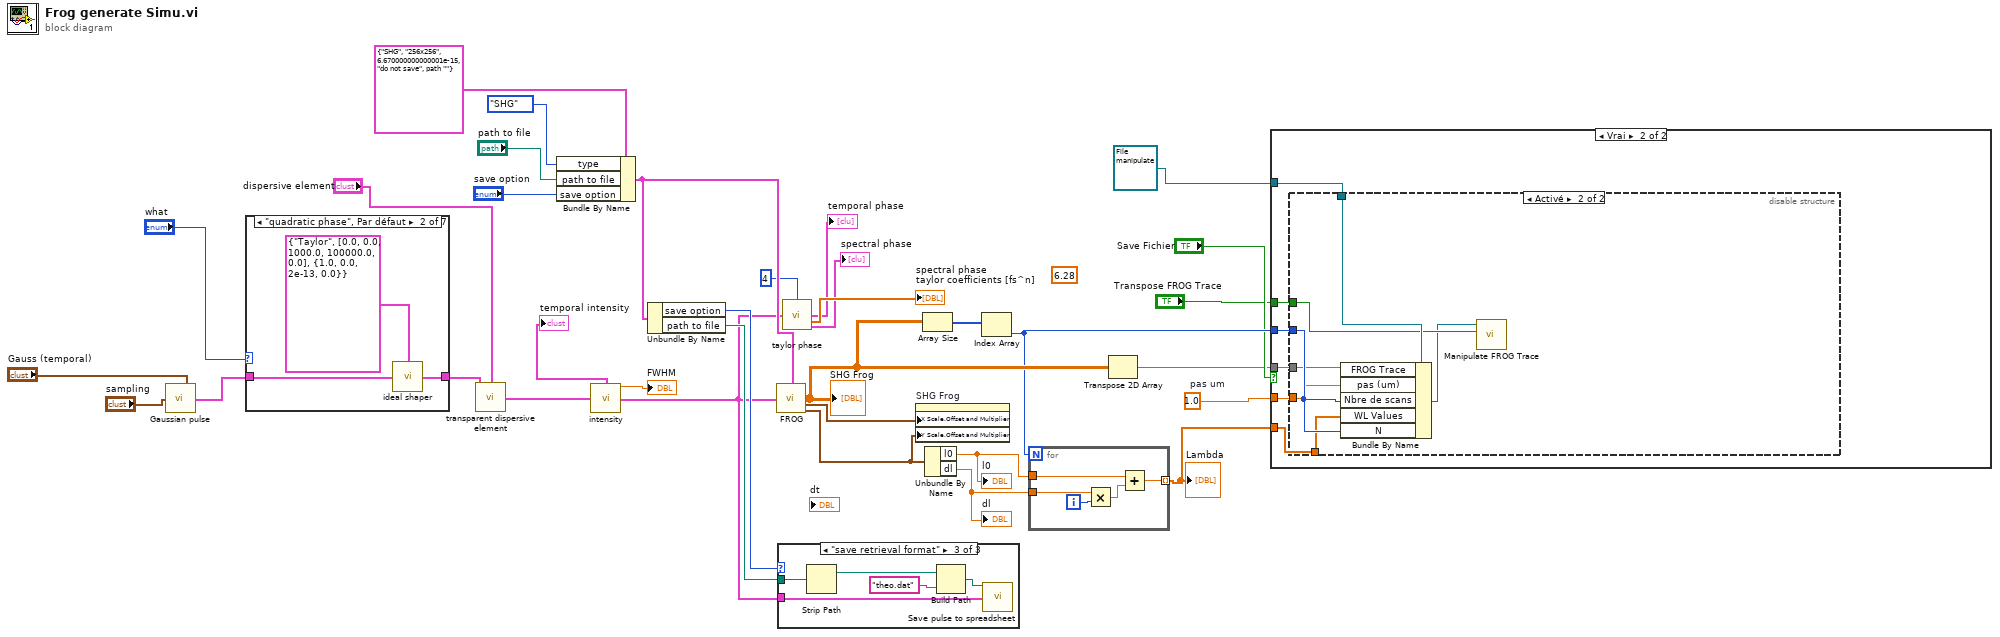
[diagram p0: block diagram]
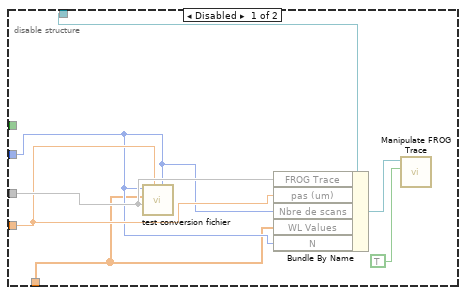
[diagram p3: hidden frame]
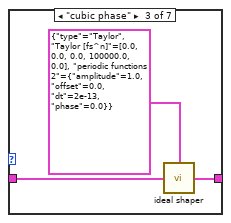
[diagram p7: hidden frame]
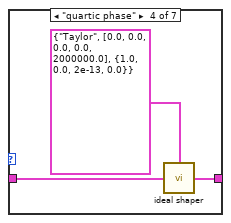
[diagram p8: hidden frame]
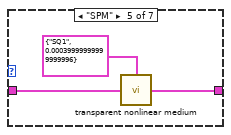
[diagram p9: hidden frame]
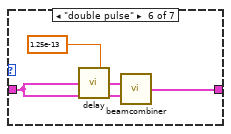
[diagram p10: hidden frame]
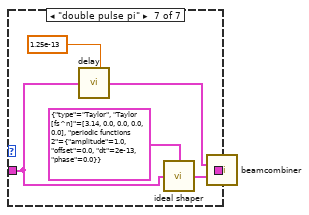
[diagram p11: hidden frame]
diagram:
  (unwired) 6.28
  w13 = 1.0  # pas um
  n1 = call <userlib>:"Gaussian pulse.vi"("Gauss (temporal)"="Gauss (temporal)", "sampling"="sampling") -> ("pulse out"=w32:T8)  [unwired: 13 in]
  n2 = case shown="\"quadratic phase\", Par défaut" "what" {
    tunnel: w32 -> [w35 w38 w41 w44 w47 w49 w54]
    tunnel: [w35 w37 w40 w43 w46 w51 w57] -> w8
    frame "no phase" {
    }
    frame "quadratic phase", Default {
      n3 = call <userlib>:"ideal shaper.vi"("phase control"=T9 {"type"=enum."Taylor", "Taylor [fs^n]"=[0.0, 0.0, 1000.0, 100000.0, 0.0], "periodic functions"={"amplitude"=1.0, "offset"=0.0, "dt"=2e-13, "phase"=0.0}}, "pulse in"=w38) -> ("pulse out"=w37:T8)  [unwired: 13 in]
    }
    frame "cubic phase" {
      n4 = call <userlib>:"ideal shaper.vi"("phase control"=T10 {"type"=enum."Taylor", "Taylor [fs^n]"=[0.0, 0.0, 0.0, 100000.0, 0.0], "periodic functions 2"={"amplitude"=1.0, "offset"=0.0, "dt"=2e-13, "phase"=0.0}}, "pulse in"=w41) -> ("pulse out"=w40:T8)  [unwired: 13 in]
    }
    frame "quartic phase" {
      n5 = call <userlib>:"ideal shaper.vi"("phase control"=T9 {"type"=enum."Taylor", "Taylor [fs^n]"=[0.0, 0.0, 0.0, 0.0, 2000000.0], "periodic functions"={"amplitude"=1.0, "offset"=0.0, "dt"=2e-13, "phase"=0.0}}, "pulse in"=w44) -> ("pulse out"=w43:T8)  [unwired: 13 in]
    }
    frame "SPM" {
      n6 = call <userlib>:"transparent nonlinear medium.vi"("nonlinear material"=cluster{"glass":string, "z":dbl[unit]} {"glass"="SQ1", "z"=0.00039999999999999996} ("nonlinear medium"), "pulse in"=w47) -> ("pulse out"=w46:T8)  [unwired: 12 in, 1 out]
    }
    frame "double pulse" {
      n7 = call <userlib>:"delay.vi"("delay time"=dbl[unit] 1.25e-13, "pulse in"=w49) -> ("pulse out"=w50:T8)  [unwired: 13 in]
      n8 = call <userlib>:"beamcombiner.vi"("pulse 1 in"=w50, "pulse 2 in"=w49) -> ("pulse out"=w51:T8)  [unwired: 13 in]
    }
    frame "double pulse pi" {
      n9 = call <userlib>:"delay.vi"("delay time"=dbl[unit] 1.25e-13, "pulse in"=w54) -> ("pulse out"=w56:T8)  [unwired: 13 in]
      n10 = call <userlib>:"ideal shaper.vi"("phase control"=T10 {"type"=enum."Taylor", "Taylor [fs^n]"=[3.14, 0.0, 0.0, 0.0, 0.0], "periodic functions 2"={"amplitude"=1.0, "offset"=0.0, "dt"=2e-13, "phase"=0.0}}, "pulse in"=w54) -> ("pulse out"=w53:T8)  [unwired: 13 in]
      n11 = call <userlib>:"beamcombiner.vi"("pulse 1 in"=w56, "pulse 2 in"=w53) -> ("pulse out"=w57:T8)  [unwired: 13 in]
    }
  }
  n12 = call <userlib>:"transparent dispersive element.vi"("dispersive element"="dispersive element", "pulse in"=w8) -> ("pulse out"=w2:T8)  [unwired: 13 in]
  n13 = Bundle By Name(cluster=T7 {"type"=enum."SHG", "field size"=enum."256x256", "time step"=6.670000000000001e-15, "save option"=enum."do not save", "path to file"=path ""} ("FROG control"), "type"=enum16{"SHG", "THG", "PG", "TG", "SD"}."SHG", "path to file"="path to file", "save option"="save option") -> (w28:T7)
  n14 = call <userlib>:"intensity.vi"("pulse in"=w2) -> ("intensity"=→"temporal intensity":T5, "FWHM t"=→"FWHM":dbl[unit], "pulse out"=w10:T8)  [unwired: 10 in, 2 out]
  n15 = Unbundle By Name(w28) -> ("save option"=w30:T4, "path to file"=w29:path)
  n16 = call <userlib>:"FROG.vi"("FROG control"=w28, "pulse in"=w10) -> ("Frog"=w17:dbl[][], "t axis"=w19:cluster{"t0":dbl, "dt":dbl}, "lambda axis"=w18:cluster{"l0":dbl, "dl":dbl})  [unwired: 11 in]
  "SHG Frog" <- w17
  n17 = case shown="\"save retrieval format\"" w30 {
    tunnel: w10 -> [_ _ w62]
    tunnel: w29 -> [_ _ w61]
    frame "do not save", Default {
    }
    frame "save jpeg" {
    }
    frame "save retrieval format" {
      n18 = Strip Path(path=w61) -> (stripped path=w60:path)  [unwired: 1 out]
      n19 = Build Path(base path=w60, name or relative path="theo.dat") -> (appended path=w59:path)
      n20 = call <userlib>:"Save pulse to spreadsheet.VI"("path"=w59, "pulse in"=w62) -> ()  [unwired: 14 in]
    }
  }
  n21 = call <userlib>:"taylor phase.vi"("order"=4, "pulse in"=w10) -> ("temporal phase"=→"temporal phase":cluster{"Y":dbl[], "Y":dbl[]}[], "spectral phase\nTaylor coefficients [fs^n]"=→"spectral phase\ntaylor coefficients [fs^n]":dbl[], "spectral phase"=→"spectral phase":cluster{"Y":dbl[], "Y":dbl[]}[])  [unwired: 10 in, 1 out]
  n22 = property on="SHG Frog" class="GraphInt (strict)"("X Scale.Offset and Multiplier"=w19, "Y Scale.Offset and Multiplier"=w18) -> ()  [unwired: 2 in, 2 out]
  n23 = Array Size(array=w17) -> (size(s)=w16:i32[])
  n24 = Unbundle By Name(w18) -> ("l0"=w15:dbl, "dl"=w14:dbl)
  "l0" <- w15
  "dl" <- w14
  n25 = Index Array(array=w16) -> (element=w12:i32)  [unwired: 1 in]
  n26 = for {
    N: w12 -> [_]
    tunnel: w15 -> [w67]
    tunnel: w14 -> [w66]
    tunnel: [w63] -> w9 mode=indexing
    i -> [w65]
    n27 = Multiply(x=w66, y=w65) -> (x*y=w64:dbl)
    n28 = Add(x=w67, y=w64) -> (x+y=w63:dbl)
  }
  "Lambda" <- w9
  n29 = Transpose 2D Array(2D array=w17) -> (transposed array=w1:dbl[][])
  n30 = case shown="Vrai" "Save Fichier" {
    tunnel: w13 -> [_ w73]
    tunnel: w12 -> [_ w72]
    tunnel: w1 -> [_ w71]
    tunnel: w9 -> [_ w70]
    tunnel: refnum<class "File manipulate.lvclass"> refnum ("File mainpulate") -> [_ w68]
    tunnel: "Transpose FROG Trace" -> [_ w69]
    frame False {
    }
    frame True {
      n31 = disable-structure shown="Activé" {
        disable-tunnel: w73 -> [w77 w83]
        disable-tunnel: w72 -> [w76 w84]
        disable-tunnel: w71 -> [w78 w81]
        disable-tunnel: w70 -> [w75 w82]
        disable-tunnel: w68 -> [w80 w87]
        disable-tunnel: w69 -> [_ w86]
        frame Disabled {
          n32 = call "test conversion fichier.vi"("Nbre de scans"=w76, "um"=w77, "FROG Trace"=w78, "WL Values"=w75, "Paramètres longueur d'onde.N"=w76) -> ()  [unwired: 1 in, 6 out]
          n33 = Bundle By Name(cluster=w80, "FROG Trace"=w78, "pas (um)"=w77, "Nbre de scans"=w76, "WL Values"=w75, "N"=w76) -> (w79:refnum<class "File manipulate.lvclass">)
          n34 = call "Manipulate FROG Trace.vi"("Transpose FROG Trace"=TRUE, "File mainpulate en entrée"=w79) -> ()  [unwired: 4 in, 6 out]
        }
        frame Enabled {
          n35 = Bundle By Name(cluster=w87, "FROG Trace"=w81, "pas (um)"=w83, "Nbre de scans"=w84, "WL Values"=w82, "N"=w84) -> (w85:refnum<class "File manipulate.lvclass">)
          n36 = call "Manipulate FROG Trace.vi"("Transpose FROG Trace"=w86, "File mainpulate en entrée"=w85) -> ()  [unwired: 4 in, 6 out]
        }
      }
    }
  }
